vi "AppendImagesToQueue.vi"(6 "Dest Format":string(combo)="{6fddc324-4e03-4bfe-b185-3d77768dc90e}", 11 "ImagesQueue":string) -> (3 "headers":string)   [LabVIEW 2016]
uses:
  <vilib>/vision/Image Controls.llb/IMAQ Image.ctl
  <vilib>/httpClient/LabVIEWHTTPClient.lvlib
panel:
  in  "password":string="gamma2018"
  in  "Remote host/IP address":string="84.253.163.35"
  in  "username":string="admin"
  out "Dest Format":string(combo)="{6fddc324-4e03-4bfe-b185-3d77768dc90e}"
  out "Image":T1(plugin-control)
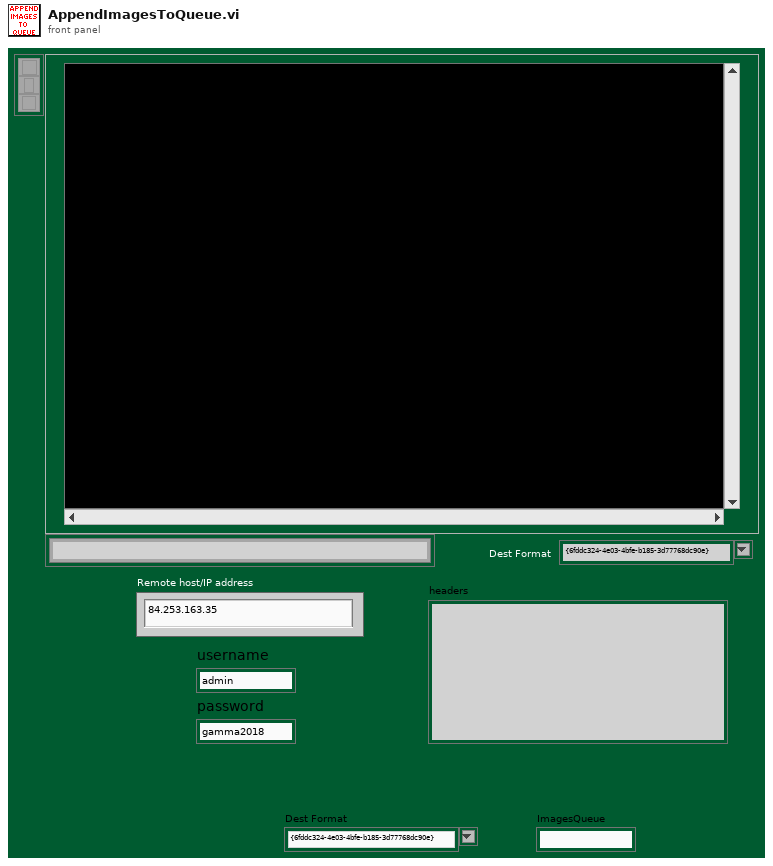
[diagram p1: front panel]
types:
  T1 = typedef "IMAQ Image.ctl" = refnum<image>
  T2 = enum16{"Show:ResetError", "Show:Exit", "Show:QueueError", "Show;Timeout_Image_Queue", "Show:Error_Imaq", "Show:Reset_Error_Recvd", "Append:Initialize", "Append:Start", "Append:Exit", "Append:QueueError", "Append:DecodeErroe", "Append:Comm not valid (Not Initialized)"}
  T3 = typedef "LabVIEWHTTPClient.lvlib/ClientHandle.ctl" = refnum<k1>
  T4 = typedef "Image Type" = u32
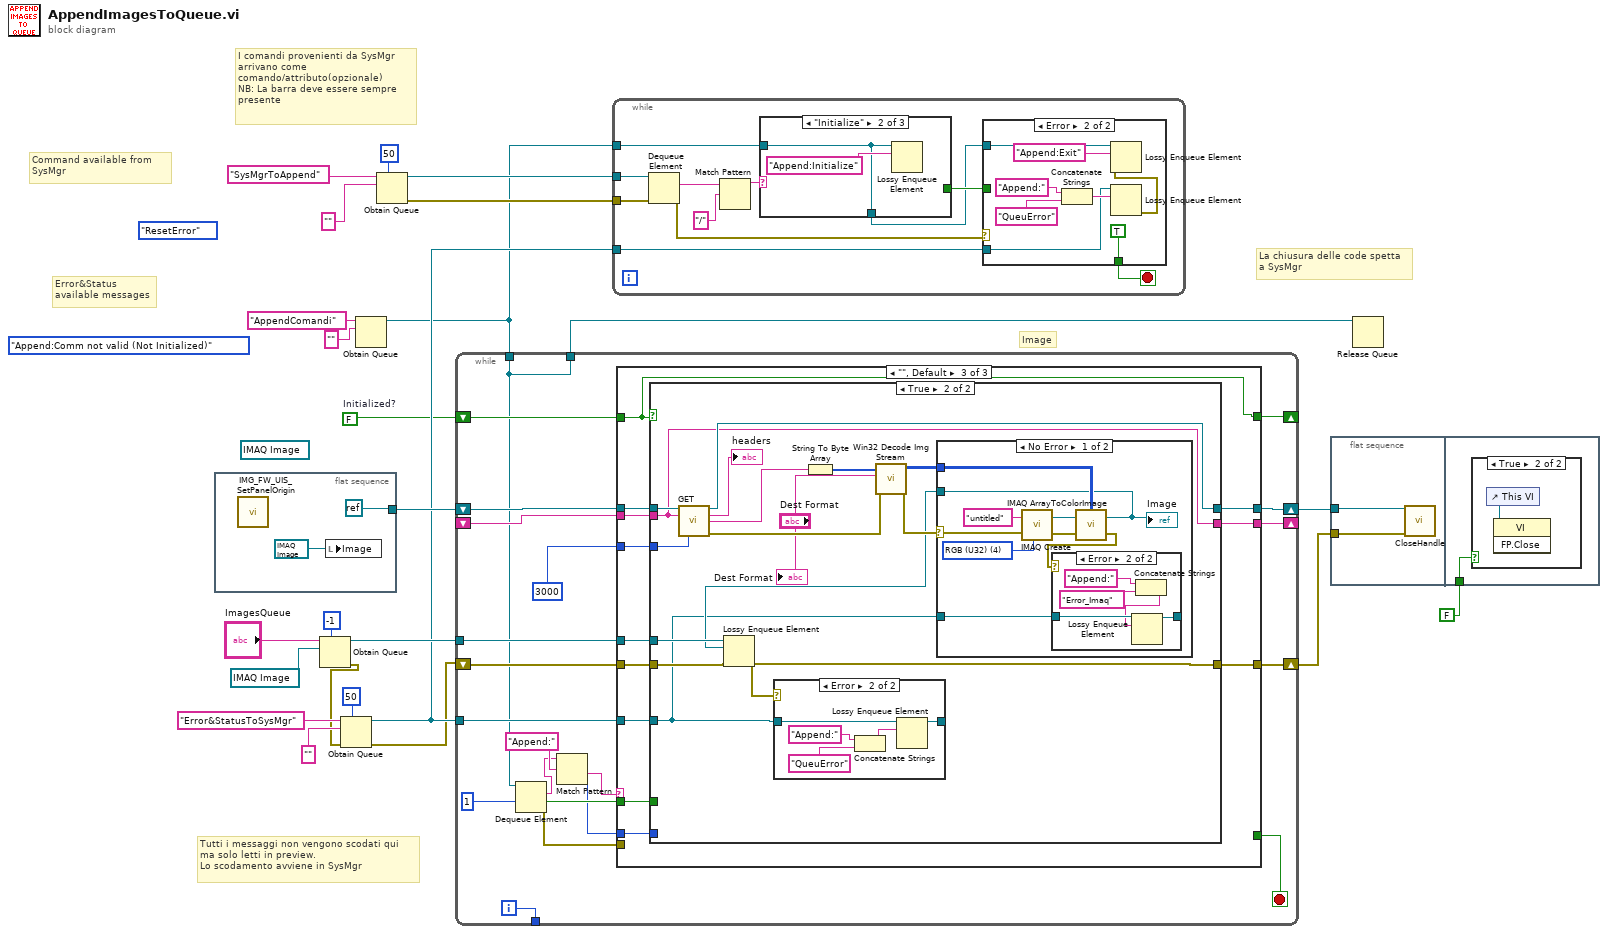
[diagram p0: block diagram]
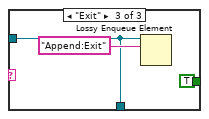
[diagram p4: hidden frame]
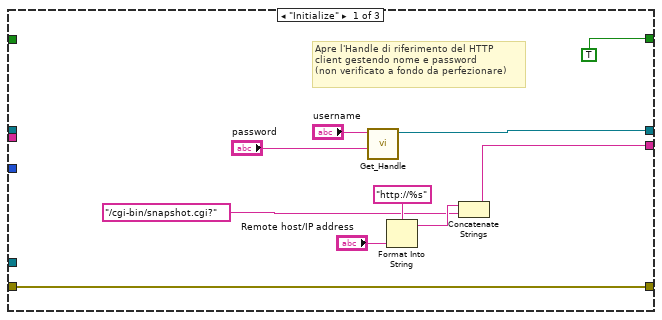
[diagram p6: hidden frame]
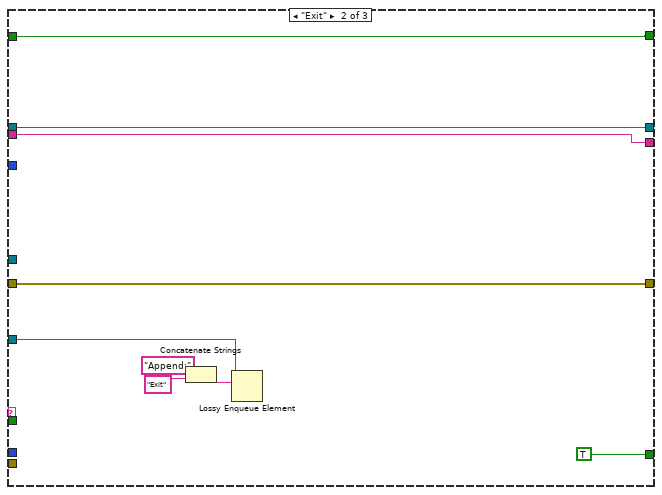
[diagram p7: hidden frame]
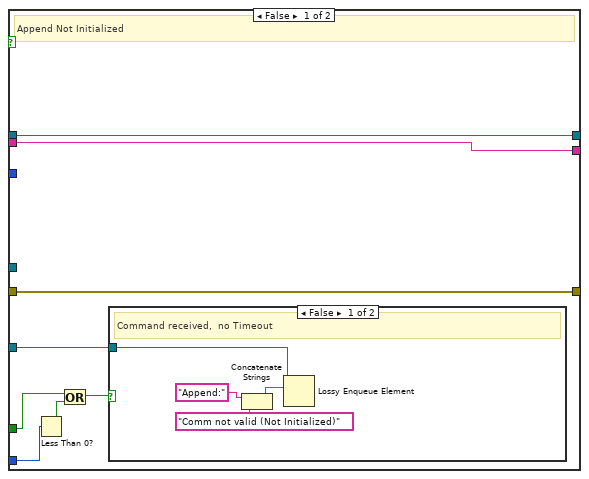
[diagram p8: hidden frame]
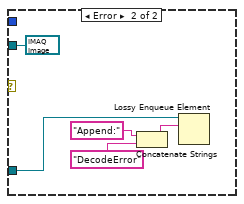
[diagram p11: hidden frame]
diagram:
  (unwired) T1 refnum ("Image")
  w9 = FALSE  # Initialized?
  (unwired) T2."Append:Comm not valid (Not Initialized)"
  (unwired) enum16{"Exit", "ResetError"}."ResetError"
  # "Image"
  # "Tutti i messaggi non vengono scodati qui\nma solo letti in preview.\nLo scodamento avviene in SysMgr"
  # "La chiusura delle code spetta\na SysMgr"
  # "I comandi provenienti da SysMgr \narrivano come\ncomando/attributo(opzionale)\nNB: La barra deve essere sempre \npresente"
  # "Error&Status\navailable messages"
  # "Command available from \nSysMgr"
  n1 = flat-sequence {
    tunnel: [refnum<k0> refnum] -> w24
    frame #0 {
      n2 = call "IMG_FW_UIS_SetPanelOrigin.vi"() -> ()  [unwired: 11 in, 1 out]
      n3 = local write "Image"(T1 refnum ("New Image")) -> ()
    }
  }
  n4 = Obtain Queue(max queue size (-1, unlimited)=-1, name (unnamed)="ImagesQueue", element data type=T1 refnum ("Image")) -> (queue out=w21:refnum<queue>, error out=w11:errorcluster)  [unwired: 2 in, 1 out]
  n5 = Obtain Queue(max queue size (-1, unlimited)=50, name (unnamed)="Error&StatusToSysMgr", element data type="", error in (no error)=w11) -> (queue out=w12:refnum<queue>, error out=w10:errorcluster)  [unwired: 1 in, 1 out]
  n6 = Obtain Queue(name (unnamed)="AppendComandi", element data type="") -> (queue out=w3:refnum<queue>)  [unwired: 3 in, 2 out]
  n7 = Obtain Queue(max queue size (-1, unlimited)=50, name (unnamed)="SysMgrToAppend", element data type="") -> (queue out=w18:refnum<queue>, error out=w20:errorcluster)  [unwired: 2 in, 1 out]
  n8 = while {
    shift-right: [w46] -> w23
    shift-left: w24 -> [w47]
    tunnel: w21 -> [w45]
    tunnel: w12 -> [w30]
    shift-right: [w33] -> w8
    shift-left: w10 -> [w44]
    shift-right: [w36] -> _
    shift-left: w9 -> [w39]
    shift-right: [w38] -> _
    shift-left: _ -> [w37]
    tunnel: [w31] -> _
    tunnel: w3 -> [w28]
    tunnel: [w28] -> w4
    i -> [w31]
    stop <- w34 stop-if-true
    n9 = Dequeue Element(queue=w28, timeout in ms (-1)=1) -> (element=w41:string, timed out?=w35:bool, error out=w29:errorcluster)  [unwired: 1 in, 1 out]
    n10 = Match Pattern(string=w41, regular expression="Append:") -> (after substring=w40:string, offset past match=w32:i32)  [unwired: 1 in, 2 out]
    n11 = case shown="\"\", Default" w40 {
      tunnel: w47 -> [_ w64 w78]
      tunnel: [w52 w64 w77] -> w46
      tunnel: w37 -> [_ w63 w76]
      tunnel: w45 -> [_ _ w75]
      tunnel: w44 -> [w48 w62 w74]
      tunnel: w39 -> [_ w65 w72]
      tunnel: [w50 w63 w71] -> w38
      tunnel: [TRUE w65 w72] -> w36
      tunnel: w35 -> [_ _ w73]
      tunnel: [_ TRUE _] -> w34
      tunnel: [w48 w62 w70] -> w33
      tunnel: w32 -> [_ _ w69]
      tunnel: w30 -> [_ w58 w68]
      tunnel: w29 -> [_ _ _]
      tunnel: u32 3000 ("millisecond multiple") -> [_ _ w67]
      frame "Initialize" {
        # "Apre l'Handle di riferimento del HTTP\nclient gestendo nome e password \n(non verificato a fondo da perfezionare)"
        n12 = call "Get_Handle.vi"("password"="password", "username"="username") -> ("Refnum out"=w52:T3)  [unwired: 9 in]
        n13 = Format Into String(format string="http://%s", "Remote host/IP address") -> (resulting string=w56:string)  [unwired: 2 in, 1 out]
        n14 = Concatenate Strings(w56, "/cgi-bin/snapshot.cgi?" ("Stringa Comando")) -> (w50:string)
      }
      frame "Exit" {
        n15 = Concatenate Strings("Append:", "Exit") -> (w59:string)
        n16 = Lossy Enqueue Element(queue=w58, element=w59) -> ()  [unwired: 1 in, 4 out]
      }
      frame "", Default {
        n17 = case shown="True" w72 {
          tunnel: w78 -> [w85 w106]
          tunnel: [w85 w96] -> w77
          tunnel: w76 -> [w86 w94]
          tunnel: w75 -> [_ w100]
          tunnel: w74 -> [w84 w99]
          tunnel: w73 -> [w82 _]
          tunnel: [w86 w94] -> w71
          tunnel: [w84 w98] -> w70
          tunnel: w69 -> [w80 _]
          tunnel: w68 -> [w79 w91]
          tunnel: w67 -> [_ w95]
          frame False {
            # "Append Not Initialized"
            n18 = Less Than 0?(x=w80) -> (x < 0?=w81:bool)
            n19 = Or(x=w82, y=w81) -> (x .or. y?=w83:bool)
            n20 = case shown="False" w83 {
              tunnel: w79 -> [w87 _]
              frame False {
                # "Command received,  no Timeout"
                n21 = Concatenate Strings("Append:", "Comm not valid (Not Initialized)") -> (w90:string)
                n22 = Lossy Enqueue Element(queue=w87, element=w90) -> ()  [unwired: 1 in, 4 out]
              }
              frame True {
                # "Timeout or no Append Command"
              }
            }
          }
          frame True {
            n23 = call <vilib>:"GET.vi"("client handle"=w106, "url"=w94, "timeout (10000)"=w95) -> ("client handle out"=w96:T3, "headers"=→"headers":string, "body"=w103:string, "error out"=w104:errorcluster)  [unwired: 9 in]
            n24 = String To Byte Array(string=w103) -> (unsigned byte array=w105:u8[])
            n25 = call "Win32 Decode Img Stream.vi"("error in (no error)"=w104, "Dest Format"="Dest Format", "Image Data"=w105) -> ("error out"=w97:errorcluster, "Dest"=w93:u32[][])  [unwired: 4 in, 3 out]
            n26 = case shown="No Error" w97 {
              selector: w97 -> [w110 _]
              tunnel: w93 -> [w111 _]
              tunnel: [w108 T1 refnum ("Image Out")] -> w92
              tunnel: w91 -> [w107 w122]
              frame No Error {
                w114 = T4 4 items=["Grayscale (U8)", "Grayscale (I16)", "Grayscale (SGL)", "Complex (CSG)", "RGB (U32)", "HSL (U32)", "RGB (U64)", "Grayscale (U16)"] ("Image Type")
                n27 = call "IMAQ Create"("Image Name"="untitled", "Image Type"=w114, "error in (no error)"=w110) -> ("New Image"=w115:T1, "error out"=w112:errorcluster)  [unwired: 2 in]
                n28 = call "IMAQ ArrayToColorImage"("Image Pixels (U32)"=w111, "Image"=w115, "error in (no error)"=w112) -> ("Image Out"=w108:T1, "error out"=w109:errorcluster)  [unwired: 2 in]
                "Image" <- w108
                n29 = case shown="Error" w109 {
                  tunnel: w107 -> [w116 w121]
                  tunnel: [w116 w118] -> _
                  frame No Error {
                  }
                  frame Error {
                    n30 = Concatenate Strings("Append:", "Error_Imaq") -> (w119:string)
                    n31 = Lossy Enqueue Element(queue=w121, element=w119) -> (queue out=w118:refnum<queue>)  [unwired: 1 in, 3 out]
                  }
                }
              }
              frame Error {
                n32 = Concatenate Strings("Append:", "DecodeError") -> (w126:string)
                n33 = Lossy Enqueue Element(queue=w122, element=w126) -> ()  [unwired: 1 in, 4 out]
              }
            }
            n34 = Lossy Enqueue Element(queue=w100, element=w92, error in (no error)=w99) -> (error out=w98:errorcluster)  [unwired: 3 out]
            n35 = case shown="Error" w98 {
              tunnel: w91 -> [w127 w130]
              tunnel: [w127 w128] -> _
              frame No Error {
              }
              frame Error {
                n36 = Concatenate Strings("Append:", "QueuError") -> (w129:string)
                n37 = Lossy Enqueue Element(queue=w130, element=w129) -> (queue out=w128:refnum<queue>)  [unwired: 1 in, 3 out]
              }
            }
            "Dest Format" <- "Dest Format"
          }
        }
      }
    }
  }
  n38 = while {
    tunnel: w18 -> [w143]
    tunnel: w20 -> [w139]
    tunnel: w12 -> [w136]
    tunnel: w3 -> [w133]
    stop <- w137 stop-if-true
    n39 = Dequeue Element(queue=w143, error in (no error)=w139) -> (element=w142:string, error out=w138:errorcluster)  [unwired: 1 in, 2 out]
    n40 = Match Pattern(string=w142, regular expression="/") -> (before substring=w140:string)  [unwired: 1 in, 3 out]
    n41 = case shown="\"Initialize\"" w140 {
      tunnel: [w153 w154 w156] -> w134
      tunnel: [_ _ TRUE] -> w135
      tunnel: w133 -> [w153 w154 w156]
      frame "", Default {
      }
      frame "Initialize" {
        n42 = Lossy Enqueue Element(queue=w154, element="Append:Initialize" ("notification")) -> ()  [unwired: 1 in, 4 out]
      }
      frame "Exit" {
        n43 = Lossy Enqueue Element(queue=w156, element="Append:Exit" ("notification")) -> ()  [unwired: 1 in, 4 out]
      }
    }
    n44 = case shown="Error" w138 {
      tunnel: [w144 TRUE] -> w137
      tunnel: w136 -> [_ w148]
      tunnel: w135 -> [w144 _]
      tunnel: w134 -> [_ w145]
      frame No Error {
      }
      frame Error {
        n45 = Concatenate Strings("Append:", "QueuError") -> (w149:string)
        n46 = Lossy Enqueue Element(queue=w148, element=w149) -> (error out=w147:errorcluster)  [unwired: 1 in, 3 out]
        n47 = Lossy Enqueue Element(queue=w145, element="Append:Exit" ("notification"), error in (no error)=w147) -> ()  [unwired: 4 out]
      }
    }
  }
  n48 = flat-sequence {
    tunnel: w8 -> [w160]
    tunnel: w23 -> [w159]
    tunnel: FALSE -> [w161]
    frame #0 {
      n49 = call <vilib>:"CloseHandle.vi"("client handle"=w159, "error in (no error)"=w160) -> ()  [unwired: 13 in, 1 out]
    }
    frame #1 {
      n50 = case shown="True" w161 {
        frame False {
        }
        frame True {
          n51 = control-ref of="This VI"() -> (w162:refnum<vi>)
          n52 = invoke class="VI" method="FP.Close"(reference=w162) -> ()  [unwired: 2 in, 3 out]
        }
      }
    }
  }
  n53 = Release Queue(queue=w4) -> ()  [unwired: 2 in, 3 out]
